vi "Dresden R2R Sputter 03.02.2018 IY24.vi"() -> ()   [LabVIEW 2009] (continued)
                                n30903 = case shown="True" w35700 {
                                frame #0 {
                                }
                                frame #1 {
                                n30904 = local write "Semi"(TRUE ("Semi")) -> ()
                                n30905 = local write "Error Message"("Coating Process cancelled.\nPlease check chamber \nconnections." ("Error Message")) -> ()
                                }
                                }
                                n30906 = local read "Ch_CC_press_ch2 2"() -> (w35694:dbl)
                                n30907 = Greater Or Equal?(x=w35694, y=5e-05 ("CHAMBER PRESSURE 5")) -> (x >= y?=w35698:bool)
                                n30908 = case shown="True" w35698 {
                                tunnel: [TRUE FALSE] -> w35697
                                frame #0 {
                                }
                                frame #1 {
                                n30909 = Wait Until Next ms Multiple(millisecond multiple=u32 200) -> ()  [unwired: 1 out]
                                }
                                }
                                n30910 = local read "Semi"() -> (w35696:bool)
                                n30911 = Or(x=w35697, y=w35696) -> (x .or. y?=w35695:bool)
                                }
                                }
                                frame #1 {
                                }
                                }
                                }
                                frame #1 {
                                n30912 = local read "Semi"() -> (w35708:bool)
                                n30913 = case shown="False" w35708 {
                                frame #0 {
                                n30914 = Wait (ms)(milliseconds to wait=u32 1000) -> ()  [unwired: 1 out]
                                n30915 = local write "SDC1 10"(TRUE ("SDC1 10")) -> ()
                                }
                                frame #1 {
                                }
                                }
                                }
                                }
                                }
                                frame #10 {
                                # "CC CLOSE"
                                n30916 = stacked-sequence {
                                frame #0 {
                                n30917 = local read "Semi"() -> (w35711:bool)
                                n30918 = case shown="False" w35711 {
                                frame #0 {
                                n30919 = while {
                                i -> [w35717]
                                stop <- w35712 stop-if-true
                                n30920 = Greater?(x=w35717, y=50) -> (0:w35716:bool)
                                n30921 = case shown="True" w35716 {
                                frame #0 {
                                }
                                frame #1 {
                                n30922 = local write "Semi"(TRUE ("Semi")) -> ()
                                n30923 = local write "Error Message"("Coating Process  \nwas cancelled.\nPlease check \nBG-BV connection." ("Error Message")) -> ()
                                }
                                }
                                n30924 = local read "Ch2_Cc_on_off_di"() -> (w35715:bool)
                                n30925 = case shown="True" w35715 {
                                tunnel: [TRUE FALSE] -> w35714
                                frame #0 {
                                }
                                frame #1 {
                                n30926 = local write "Ch2_Cc_on_off_do"(FALSE ("Ch1_WFC_do")) -> ()
                                n30927 = Wait Until Next ms Multiple(millisecond multiple=u32 200) -> ()  [unwired: 1 out]
                                }
                                }
                                n30928 = local read "Semi"() -> (w35713:bool)
                                n30929 = Or(x=w35714, y=w35713) -> (x .or. y?=w35712:bool)
                                }
                                }
                                frame #1 {
                                }
                                }
                                }
                                frame #1 {
                                n30930 = local read "Semi"() -> (w35725:bool)
                                n30931 = case shown="False" w35725 {
                                frame #0 {
                                n30932 = local write "SDC1 10b"(TRUE ("SDC1 3")) -> ()
                                n30933 = Wait (ms)(milliseconds to wait=u32 1000) -> ()  [unwired: 1 out]
                                }
                                frame #1 {
                                }
                                }
                                }
                                }
                                }
                                frame #11 {
                                # "DC -Ignite Plasma"
                                n30934 = stacked-sequence {
                                frame #0 {
                                n30935 = local read "Semi"() -> (w35728:bool)
                                n30936 = case shown="False" w35728 {
                                frame #0 {
                                n30937 = stacked-sequence {
                                frame #0 {
                                n30938 = local read "Semi"() -> (w35729:bool)
                                n30939 = case shown="False" w35729 {
                                frame #0 {
                                n30940 = while {
                                i -> [w35735]
                                stop <- w35730 stop-if-true
                                n30941 = Greater?(x=w35735, y=50) -> (0:w35734:bool)
                                n30942 = case shown="True" w35734 {
                                frame #0 {
                                }
                                frame #1 {
                                n30943 = local write "Semi"(TRUE ("Semi")) -> ()
                                n30944 = local write "Error Message"("Sputtering Process cancelled.\nPlease check \nDC switch connections." ("Error Message")) -> ()
                                }
                                }
                                n30945 = local read "Cnt_Dcps_sw2_di"() -> (w35733:bool)
                                n30946 = case shown="True" w35733 {
                                tunnel: [TRUE ("Cnt_Dcps_sw1_do") FALSE ("Cnt_Dcps_sw1_do")] -> w35732
                                frame #0 {
                                }
                                frame #1 {
                                n30947 = local write "Cnt_Dcps_sw2_do"(FALSE ("Cnt_Dcps_sw1_do")) -> ()
                                n30948 = Wait Until Next ms Multiple(millisecond multiple=u32 200) -> ()  [unwired: 1 out]
                                }
                                }
                                n30949 = local read "Semi"() -> (w35731:bool)
                                n30950 = Or(x=w35732, y=w35731) -> (x .or. y?=w35730:bool)
                                }
                                }
                                frame #1 {
                                }
                                }
                                }
                                frame #1 {
                                n30951 = local read "Semi"() -> (w35743:bool)
                                n30952 = case shown="False" w35743 {
                                frame #0 {
                                n30953 = while {
                                i -> [w35749]
                                stop <- w35744 stop-if-true
                                n30954 = Greater?(x=w35749, y=50) -> (0:w35748:bool)
                                n30955 = case shown="True" w35748 {
                                frame #0 {
                                }
                                frame #1 {
                                n30956 = local write "Semi"(TRUE ("Semi")) -> ()
                                n30957 = local write "Error Message"("Sputtering Process cancelled.\nPlease check \nDC switch connections." ("Error Message")) -> ()
                                }
                                }
                                n30958 = local read "Cnt_Dcps_sw1_di"() -> (w35747:bool)
                                n30959 = case shown="False" w35747 {
                                tunnel: [FALSE ("Cnt_Dcps_sw1_do") TRUE ("Cnt_Dcps_sw1_do")] -> w35746
                                frame #0 {
                                n30960 = local write "Cnt_Dcps_sw1_do"(TRUE ("Cnt_Dcps_sw1_do")) -> ()
                                n30961 = Wait Until Next ms Multiple(millisecond multiple=u32 200) -> ()  [unwired: 1 out]
                                }
                                frame #1 {
                                }
                                }
                                n30962 = local read "Semi"() -> (w35745:bool)
                                n30963 = Or(x=w35746, y=w35745) -> (x .or. y?=w35744:bool)
                                }
                                }
                                frame #1 {
                                }
                                }
                                }
                                frame #2 {
                                n30964 = local read "Semi"() -> (w35757:bool)
                                n30965 = case shown="False" w35757 {
                                frame #0 {
                                n30966 = local write "Dc_host_auto"(TRUE ("Dc_host_auto")) -> ()
                                }
                                frame #1 {
                                }
                                }
                                }
                                frame #3 {
                                n30967 = local read "Semi"() -> (w35759:bool)
                                n30968 = case shown="False" w35759 {
                                frame #0 {
                                n30969 = local read "R Cmb Ch2 Step1 Coating Power Active"() -> (w35770:bool)
                                n30970 = local read "R Cmb Ch2 Step2 Coating Power Active"() -> (w35769:bool)
                                n30971 = local read "R Cmb Ch2 Step3 Coating Power Active"() -> (w35768:bool)
                                n30972 = local read "R Cmb Ch2 Step4 Coating Power Active"() -> (w35767:bool)
                                n30973 = local read "R Cmb Ch2 Step5 Coating Power Active"() -> (w35766:bool)
                                n30974 = Boolean To (0,1)(Boolean=w35770) -> (0, 1=w35765:i16)
                                n30975 = Boolean To (0,1)(Boolean=w35769) -> (0, 1=w35764:i16)
                                n30976 = Boolean To (0,1)(Boolean=w35768) -> (0, 1=w35763:i16)
                                n30977 = Boolean To (0,1)(Boolean=w35767) -> (0, 1=w35762:i16)
                                n30978 = Boolean To (0,1)(Boolean=w35766) -> (0, 1=w35761:i16)
                                n30979 = Compound Arithmetic op=ADD(w35765, w35764, w35763, w35762, w35761) -> (w35760:i16)
                                n30980 = case shown="0, Default" w35760 {
                                frame #0 {
                                }
                                frame #1 {
                                n30981 = local read "R Cmb Ch2 Step1 Coating Power"() -> (w35771:dbl)
                                n30982 = local write "Set DC Power       :"(w35771) -> ()
                                }
                                frame #2 {
                                n30983 = local read "R Cmb Ch2 Step2 Coating Power"() -> (w35772:dbl)
                                n30984 = local write "Set DC Power       :"(w35772) -> ()
                                }
                                frame #3 {
                                n30985 = local read "R Cmb Ch2 Step3 Coating Power"() -> (w35773:dbl)
                                n30986 = local write "Set DC Power       :"(w35773) -> ()
                                }
                                frame #4 {
                                n30987 = local read "R Cmb Ch2 Step4 Coating Power"() -> (w35774:dbl)
                                n30988 = local write "Set DC Power       :"(w35774) -> ()
                                }
                                frame #5 {
                                n30989 = local read "R Cmb Ch2 Step5 Coating Power"() -> (w35775:dbl)
                                n30990 = local write "Set DC Power       :"(w35775) -> ()
                                }
                                }
                                }
                                frame #1 {
                                }
                                }
                                }
                                frame #4 {
                                n30991 = local read "Semi"() -> (w35776:bool)
                                n30992 = case shown="False" w35776 {
                                frame #0 {
                                n30993 = Wait (ms)(milliseconds to wait=u32 1000) -> ()  [unwired: 1 out]
                                }
                                frame #1 {
                                }
                                }
                                }
                                frame #5 {
                                n30994 = local read "Semi"() -> (w35778:bool)
                                n30995 = case shown="False" w35778 {
                                frame #0 {
                                n30996 = local write "Dc_auto_set"(TRUE ("Dc_auto_set")) -> ()
                                }
                                frame #1 {
                                }
                                }
                                }
                                frame #6 {
                                n30997 = local read "Semi"() -> (w35780:bool)
                                n30998 = case shown="False" w35780 {
                                frame #0 {
                                n30999 = Wait (ms)(milliseconds to wait=u32 1000) -> ()  [unwired: 1 out]
                                }
                                frame #1 {
                                }
                                }
                                }
                                }
                                }
                                frame #1 {
                                }
                                }
                                }
                                frame #1 {
                                n31000 = local read "Semi"() -> (w35782:bool)
                                n31001 = case shown="False" w35782 {
                                frame #0 {
                                n31002 = Wait (ms)(milliseconds to wait=u32 1000) -> ()  [unwired: 1 out]
                                n31003 = local write "SDC1 13"(TRUE ("SDC1 13")) -> ()
                                }
                                frame #1 {
                                }
                                }
                                }
                                }
                                }
                                frame #12 {
                                n31004 = local read "Web_selection_tab"() -> (w35785:T5)
                                n31005 = case shown="\"Web                                                                                    \", Default" w35785 {
                                frame #0 {
                                n31006 = stacked-sequence {
                                frame #0 {
                                n31007 = local read "R Web speed(cm/min)"() -> (w35788:dbl)
                                n31008 = local read "R Maximum diameter"() -> (w35786:dbl)
                                n31009 = local read "R Web thicness"() -> (w35787:dbl)
                                n31010 = Wait (ms)(milliseconds to wait=u32 1000) -> ()  [unwired: 1 out]
                                n31011 = local write "Change_Max Diameter"(w35786) -> ()
                                n31012 = local write "Web Thickness"(w35787) -> ()
                                n31013 = local write "Web Speed"(w35788) -> ()
                                }
                                frame #1 {
                                n31014 = local write "Calculate 3"(TRUE ("Calculate 3")) -> ()
                                }
                                frame #2 {
                                n31015 = local read "Change_Max Diameter"() -> (w35792:dbl)
                                n31016 = Wait (ms)(milliseconds to wait=u32 1000) -> ()  [unwired: 1 out]
                                n31017 = local write "Initial Min Diameter"(w35792) -> ()
                                }
                                frame #3 {
                                n31018 = local read "R Cmb Ch2 Step1 Coating Power Active"() -> (w35793:bool)
                                n31019 = local read "R Cmb Ch2 Step2 Coating Power Active"() -> (w35794:bool)
                                n31020 = local read "R Cmb Ch2 Step3 Coating Power Active"() -> (w35795:bool)
                                n31021 = local read "R Cmb Ch2 Step4 Coating Power Active"() -> (w35796:bool)
                                n31022 = local read "R Cmb Ch2 Step5 Coating Power Active"() -> (w35797:bool)
                                n31023 = Boolean To (0,1)(Boolean=w35793) -> (0, 1=w35798:i16)
                                n31024 = Boolean To (0,1)(Boolean=w35794) -> (0, 1=w35799:i16)
                                n31025 = Boolean To (0,1)(Boolean=w35795) -> (0, 1=w35800:i16)
                                n31026 = Boolean To (0,1)(Boolean=w35796) -> (0, 1=w35801:i16)
                                n31027 = Boolean To (0,1)(Boolean=w35797) -> (0, 1=w35802:i16)
                                n31028 = Compound Arithmetic op=ADD(w35798, w35799, w35800, w35801, w35802) -> (w35804:i16)
                                n31029 = Wait (ms)(milliseconds to wait=u32 200) -> ()  [unwired: 1 out]
                                n31030 = local read "R Cmb Interval length"() -> (w35803:dbl)
                                n31031 = Multiply(x=w35803, y=w35804) -> (x*y=w35805:dbl)
                                n31032 = local write "Total length"(w35805) -> ()
                                }
                                frame #4 {
                                n31033 = local write "Calculate 2"(TRUE ("Calculate_auto")) -> ()
                                }
                                frame #5 {
                                n31034 = Wait (ms)(milliseconds to wait=u32 1000) -> ()  [unwired: 1 out]
                                n31035 = local write "Roll_side_select"(enum32{"Left to Right", "Right to Left"}."Right to Left" ("Roll_side_select")) -> ()
                                }
                                frame #6 {
                                n31036 = Wait (ms)(milliseconds to wait=u32 100) -> ()  [unwired: 1 out]
                                n31037 = local write "Parameters_auto_set"(TRUE ("Parameters_auto_set")) -> ()
                                }
                                frame #7 {
                                n31038 = while {
                                i -> [w35816]
                                stop <- w35812 stop-if-true
                                n31039 = Wait Until Next ms Multiple(millisecond multiple=u32 300) -> ()  [unwired: 1 out]
                                n31040 = Greater?(x=w35816, y=100) -> (0:w35813:bool)
                                n31041 = local read "Parameters_auto_set"() -> (w35817:bool)
                                n31042 = case shown="False" w35817 {
                                tunnel: [TRUE FALSE] -> w35814
                                frame #0 {
                                }
                                frame #1 {
                                }
                                }
                                n31043 = Or(x=w35814, y=w35813) -> (x .or. y?=w35812:bool)
                                }
                                }
                                frame #8 {
                                n31044 = local read "R Tension Value"() -> (w35821:dbl)
                                n31045 = Wait (ms)(milliseconds to wait=u32 200) -> ()  [unwired: 1 out]
                                n31046 = local write "TC2_set_value"(w35821) -> ()
                                }
                                frame #9 {
                                n31047 = local write "TC2_auto_set"(TRUE ("TC1_auto_set")) -> ()
                                }
                                frame #10 {
                                w35825 = u16 1 items=["1", "2", "3", "4"] ("Target Chamber Sensor")
                                n31048 = local write "Target Chamber Sensor"(w35825) -> ()
                                n31049 = Wait (ms)(milliseconds to wait=u32 200) -> ()  [unwired: 1 out]
                                }
                                frame #11 {
                                n31050 = local read "Total length"() -> (w35827:dbl)
                                n31051 = Wait (ms)(milliseconds to wait=u32 100) -> ()  [unwired: 1 out]
                                n31052 = local write "Region"(w35827) -> ()
                                }
                                frame #12 {
                                n31053 = local read "Semi"() -> (w35828:bool)
                                n31054 = case shown="False" w35828 {
                                frame #0 {
                                n31055 = stacked-sequence {
                                frame #0 {
                                # "Gas Flow"
                                n31056 = stacked-sequence {
                                frame #0 {
                                n31057 = local read "Semi"() -> (w35829:bool)
                                n31058 = case shown="False" w35829 {
                                frame #0 {
                                n31059 = stacked-sequence {
                                frame #0 {
                                n31060 = local read "Semi"() -> (w35830:bool)
                                n31061 = case shown="False" w35830 {
                                frame #0 {
                                n31062 = local read "R Argon Flow sccm"() -> (w35831:dbl)
                                n31063 = local write "Ar_sccm1_2"(w35831) -> ()
                                }
                                frame #1 {
                                }
                                }
                                }
                                frame #1 {
                                n31064 = local read "Semi"() -> (w35832:bool)
                                n31065 = case shown="False" w35832 {
                                frame #0 {
                                n31066 = local write "Mfc_Ar _1_2_set"(TRUE ("Mfc_Ar _1_2_set")) -> ()
                                }
                                frame #1 {
                                }
                                }
                                }
                                frame #2 {
                                n31067 = local read "Semi"() -> (w35834:bool)
                                n31068 = case shown="False" w35834 {
                                frame #0 {
                                n31069 = while {
                                i -> [w35837]
                                stop <- w35839 stop-if-true
                                n31070 = Greater?(x=w35837, y=50) -> (0:w35836:bool)
                                n31071 = local read "Semi"() -> (w35835:bool)
                                n31072 = Or(x=w35835, y=w35836) -> (x .or. y?=w35839:bool)
                                }
                                }
                                frame #1 {
                                }
                                }
                                }
                                frame #3 {
                                n31073 = local read "Semi"() -> (w35840:bool)
                                n31074 = case shown="False" w35840 {
                                frame #0 {
                                n31075 = local read "Ar_sccm_act 6"() -> (w35841:dbl)
                                n31076 = Greater?(x=w35841, y=1) -> (0:w35842:bool)
                                n31077 = case shown="False" w35842 {
                                frame #0 {
                                n31078 = local read "R Argon Flow sccm"() -> (w35844:dbl)
                                n31079 = local write "Ar_sccm1_2"(w35844) -> ()
                                }
                                frame #1 {
                                }
                                }
                                }
                                frame #1 {
                                }
                                }
                                }
                                frame #4 {
                                n31080 = local read "Semi"() -> (w35845:bool)
                                n31081 = case shown="False" w35845 {
                                frame #0 {
                                n31082 = local read "Ar_sccm_act 6"() -> (w35847:dbl)
                                n31083 = Greater?(x=w35847, y=1) -> (0:w35846:bool)
                                n31084 = case shown="False" w35846 {
                                frame #0 {
                                n31085 = while {
                                i -> [w35850]
                                stop <- w35854 stop-if-true
                                n31086 = Greater?(x=w35850, y=50) -> (0:w35849:bool)
                                n31087 = local read "Semi"() -> (w35853:bool)
                                n31088 = case shown="False" w35853 {
                                tunnel: [FALSE TRUE] -> w35852
                                frame #0 {
                                n31089 = Wait Until Next ms Multiple(millisecond multiple=u32 200) -> ()  [unwired: 1 out]
                                }
                                frame #1 {
                                }
                                }
                                n31090 = Or(x=w35852, y=w35849) -> (x .or. y?=w35854:bool)
                                }
                                }
                                frame #1 {
                                }
                                }
                                }
                                frame #1 {
                                }
                                }
                                }
                                frame #5 {
                                n31091 = local read "Semi"() -> (w35858:bool)
                                n31092 = case shown="False" w35858 {
                                frame #0 {
                                n31093 = local read "Ar_sccm_act 5"() -> (w35860:dbl)
                                n31094 = Greater?(x=w35860, y=1) -> (0:w35859:bool)
                                n31095 = case shown="False" w35859 {
                                frame #0 {
                                n31096 = local write "Semi"(TRUE ("Semi")) -> ()
                                n31097 = local write "Error Message"("Coating process cancelled.\nPlease check connections." ("Error Message")) -> ()
                                }
                                frame #1 {
                                }
                                }
                                }
                                frame #1 {
                                }
                                }
                                }
                                }
                                }
                                frame #1 {
                                }
                                }
                                }
                                frame #1 {
                                n31098 = local read "Semi"() -> (w35864:bool)
                                n31099 = case shown="False" w35864 {
                                frame #0 {
                                n31100 = local write "SDC1 11"(TRUE ("SDC1 11")) -> ()
                                n31101 = Wait (ms)(milliseconds to wait=u32 1000) -> ()  [unwired: 1 out]
                                }
                                frame #1 {
                                }
                                }
                                }
                                }
                                }
                                frame #1 {
                                # "Set Pressure for ignite plasma"
                                n31102 = stacked-sequence {
                                frame #0 {
                                n31103 = local read "Semi"() -> (w35867:bool)
                                n31104 = case shown="False" w35867 {
                                frame #0 {
                                n31105 = stacked-sequence {
                                frame #0 {
                                n31106 = local read "Semi"() -> (w35868:bool)
                                n31107 = case shown="False" w35868 {
                                frame #0 {
                                n31108 = local write "Set_pressure_value 2"(10.0 ("Set_pressure_value 2")) -> ()
                                }
                                frame #1 {
                                }
                                }
                                }
                                frame #1 {
                                n31109 = local read "Semi"() -> (w35870:bool)
                                n31110 = case shown="False" w35870 {
                                frame #0 {
                                n31111 = Wait (ms)(milliseconds to wait=u32 1000) -> ()  [unwired: 1 out]
                                }
                                frame #1 {
                                }
                                }
                                }
                                frame #2 {
                                n31112 = local read "Semi"() -> (w35872:bool)
                                n31113 = case shown="False" w35872 {
                                frame #0 {
                                n31114 = local write "Pc_bv2_auto_set_pressure"(TRUE ("Pc_bv1_auto_set_pressure")) -> ()
                                }
                                frame #1 {
                                }
                                }
                                }
                                frame #3 {
                                n31115 = local read "Semi"() -> (w35874:bool)
                                n31116 = case shown="False" w35874 {
                                frame #0 {
                                n31117 = while {
                                i -> [w35885]
                                stop <- w35877 stop-if-true
                                w35875 = 10.0 ("Set_pressure_value 2")
                                n31118 = Greater?(x=w35885, y=300) -> (0:w35879:bool)
                                n31119 = Add(x=1.0, y=w35875) -> (x+y=w35881:dbl)
                                n31120 = Subtract(x=w35875, y=1.0) -> (x-y=w35882:dbl)
                                n31121 = local read "Pressure 2"() -> (w35876:i32)
                                n31122 = In Range and Coerce(upper limit=w35881, x=w35876, lower limit=w35882) -> (In Range?=w35880:bool)  [unwired: 1 out]
                                n31123 = case shown="False" w35880 {
                                tunnel: [FALSE TRUE] -> w35878
                                frame #0 {
                                n31124 = Wait Until Next ms Multiple(millisecond multiple=u32 200) -> ()  [unwired: 1 out]
                                }
                                frame #1 {
                                }
                                }
                                n31125 = Or(x=w35878, y=w35879) -> (x .or. y?=w35877:bool)
                                }
                                }
                                frame #1 {
                                }
                                }
                                }
                                frame #4 {
                                n31126 = local read "Semi"() -> (w35890:bool)
                                n31127 = case shown="False" w35890 {
                                frame #0 {
                                w35891 = 10.0 ("Set_pressure_value 2")
                                n31128 = Add(x=1.0, y=w35891) -> (x+y=w35894:dbl)
                                n31129 = Subtract(x=w35891, y=1.0) -> (x-y=w35895:dbl)
                                n31130 = local read "Pressure 2"() -> (w35892:i32)
                                n31131 = In Range and Coerce(upper limit=w35894, x=w35892, lower limit=w35895) -> (In Range?=w35893:bool)  [unwired: 1 out]
                                n31132 = case shown="False" w35893 {
                                frame #0 {
                                n31133 = local read "R Set Pressure mtorr"() -> (w35898:dbl)
                                n31134 = local write "Set_pressure_value 2"(w35898) -> ()
                                }
                                frame #1 {
                                }
                                }
                                }
                                frame #1 {
                                }
                                }
                                }
                                frame #5 {
                                n31135 = local read "Semi"() -> (w35899:bool)
                                n31136 = case shown="False" w35899 {
                                frame #0 {
                                w35900 = 10.0 ("Set_pressure_value 2")
                                n31137 = Add(x=1.0, y=w35900) -> (x+y=w35903:dbl)
                                n31138 = Subtract(x=w35900, y=1.0) -> (x-y=w35904:dbl)
                                n31139 = local read "Pressure 2"() -> (w35901:i32)
                                n31140 = In Range and Coerce(upper limit=w35903, x=w35901, lower limit=w35904) -> (In Range?=w35902:bool)  [unwired: 1 out]
                                n31141 = case shown="False" w35902 {
                                frame #0 {
                                n31142 = local write "Pc_bv2_auto_set_pressure"(TRUE ("Pc_bv1_auto_set_pressure")) -> ()
                                }
                                frame #1 {
                                }
                                }
                                }
                                frame #1 {
                                }
                                }
                                }
                                frame #6 {
                                n31143 = local read "Semi"() -> (w35908:bool)
                                n31144 = case shown="False" w35908 {
                                frame #0 {
                                n31145 = while {
                                i -> [w35919]
                                stop <- w35911 stop-if-true
                                w35909 = 10.0 ("Set_pressure_value 2")
                                n31146 = Greater?(x=w35919, y=300) -> (0:w35913:bool)
                                n31147 = Add(x=1.0, y=w35909) -> (x+y=w35915:dbl)
                                n31148 = Subtract(x=w35909, y=1.0) -> (x-y=w35916:dbl)
                                n31149 = local read "Pressure 2"() -> (w35910:i32)
                                n31150 = In Range and Coerce(upper limit=w35915, x=w35910, lower limit=w35916) -> (In Range?=w35914:bool)  [unwired: 1 out]
                                n31151 = case shown="False" w35914 {
                                tunnel: [FALSE TRUE] -> w35912
                                frame #0 {
                                n31152 = Wait Until Next ms Multiple(millisecond multiple=u32 200) -> ()  [unwired: 1 out]
                                }
                                frame #1 {
                                }
                                }
                                n31153 = Or(x=w35912, y=w35913) -> (x .or. y?=w35911:bool)
                                }
                                }
                                frame #1 {
                                }
                                }
                                }
                                frame #7 {
                                n31154 = local read "Semi"() -> (w35924:bool)
                                n31155 = case shown="False" w35924 {
                                frame #0 {
                                n31156 = local read "Set_pressure_value 2"() -> (w35927:dbl)
                                n31157 = Add(x=1.0, y=w35927) -> (x+y=w35928:dbl)
                                n31158 = Subtract(x=w35927, y=1.0) -> (x-y=w35929:dbl)
                                n31159 = local read "Pressure 2"() -> (w35925:i32)
                                n31160 = In Range and Coerce(upper limit=w35928, x=w35925, lower limit=w35929) -> (In Range?=w35926:bool)  [unwired: 1 out]
                                n31161 = case shown="False" w35926 {
                                frame #0 {
                                n31162 = local write "Semi"(TRUE ("Semi")) -> ()
                                n31163 = local write "Error Message"("Coating Pressure could not be adjusted !" ("Error Message")) -> ()
                                }
                                frame #1 {
                                }
                                }
                                }
                                frame #1 {
                                }
                                }
                                }
                                }
                                }
                                frame #1 {
                                }
                                }
                                }
                                frame #1 {
                                n31164 = local read "Semi"() -> (w35934:bool)
                                n31165 = case shown="False" w35934 {
                                frame #0 {
                                n31166 = local write "SDC1 9"(TRUE ("SDC1 9")) -> ()
                                n31167 = Wait (ms)(milliseconds to wait=u32 1000) -> ()  [unwired: 1 out]
                                }
                                frame #1 {
                                }
                                }
                                }
                                }
                                }
                                frame #2 {
                                # "Plasma ignite and check"
                                n31168 = stacked-sequence {
                                frame #0 {
                                n31169 = local read "Semi"() -> (w35937:bool)
                                n31170 = case shown="False" w35937 {
                                frame #0 {
                                n31171 = local write "Dc_auto_on"(TRUE ("Dc_auto_on")) -> ()
                                }
                                frame #1 {
                                }
                                }
                                }
                                frame #1 {
                                n31172 = local read "Semi"() -> (w35939:bool)
                                n31173 = case shown="False" w35939 {
                                frame #0 {
                                n31174 = while {
                                i -> [w35949]
                                stop <- w35940 stop-if-true
                                n31175 = Greater Or Equal?(x=w35949, y=240) -> (x >= y?=w35948:bool)
                                n31176 = case shown="True" w35948 {
                                frame #0 {
                                }
                                frame #1 {
                                n31177 = local write "Semi"(TRUE ("Semi")) -> ()
                                }
                                }
                                n31178 = local read "Set DC Power       :"() -> (w35945:dbl)
                                n31179 = local read "Actual DC Power"() -> (w35944:dbl)
                                n31180 = Subtract(x=w35945, y=w35944) -> (x-y=w35947:dbl)
                                n31181 = Less?(x=w35947, y=10.0) -> (x < y?=w35942:bool)
                                n31182 = local read "Semi"() -> (w35941:bool)
                                n31183 = Or(x=w35942, y=w35941) -> (x .or. y?=w35940:bool)
                                n31184 = Wait Until Next ms Multiple(millisecond multiple=u32 500) -> ()  [unwired: 1 out]
                                }
                                }
                                frame #1 {
                                }
                                }
                                }
                                }
                                }
                                frame #3 {
                                # "Set Pressure for coating"
                                n31185 = stacked-sequence {
                                frame #0 {
                                n31186 = local read "Semi"() -> (w35952:bool)
                                n31187 = case shown="False" w35952 {
                                frame #0 {
                                n31188 = stacked-sequence {
                                frame #0 {
                                n31189 = local read "Semi"() -> (w35953:bool)
                                n31190 = case shown="False" w35953 {
                                frame #0 {
                                n31191 = local read "R Set Pressure mtorr"() -> (w35954:dbl)
                                n31192 = local write "Set_pressure_value 2"(w35954) -> ()
                                }
                                frame #1 {
                                }
                                }
                                }
                                frame #1 {
                                n31193 = local read "Semi"() -> (w35955:bool)
                                n31194 = case shown="False" w35955 {
                                frame #0 {
                                n31195 = Wait (ms)(milliseconds to wait=u32 200) -> ()  [unwired: 1 out]
                                }
                                frame #1 {
                                }
                                }
                                }
                                frame #2 {
                                n31196 = local read "Semi"() -> (w35957:bool)
                                n31197 = case shown="False" w35957 {
                                frame #0 {
                                n31198 = local write "Pc_bv2_auto_set_pressure"(TRUE ("Pc_bv1_auto_set_pressure")) -> ()
                                }
                                frame #1 {
                                }
                                }
                                }
                                frame #3 {
                                n31199 = local read "Semi"() -> (w35959:bool)
                                n31200 = case shown="False" w35959 {
                                frame #0 {
                                n31201 = while {
                                i -> [w35970]
                                stop <- w35962 stop-if-true
                                n31202 = local read "Set_pressure_value 2"() -> (w35960:dbl)
                                n31203 = Greater?(x=w35970, y=300) -> (0:w35964:bool)
                                n31204 = Add(x=1.0, y=w35960) -> (x+y=w35966:dbl)
                                n31205 = Subtract(x=w35960, y=1.0) -> (x-y=w35967:dbl)
                                n31206 = local read "Pressure 2"() -> (w35961:i32)
                                n31207 = In Range and Coerce(upper limit=w35966, x=w35961, lower limit=w35967) -> (In Range?=w35965:bool)  [unwired: 1 out]